vi "BuildThermomechanicalStave-Old.vi"() -> ()   [LabVIEW 2016]
doc: "This VI is the overarching framework for the ITk Stave Assembly at Brookhaven National Lab. This VI coordinates all SubVIs so that the user can execute all phases of construction: Calibration, Module Placement, and Final Survey. Learn more at https://github.com/sciollalab/BNL_ThermomechanicalStave/wiki"
uses:
  <vilib>/userdefined/High Color/IMAQdx.ctl
  Utils/Controls/All_Enums/Enum_TypeDef_CameraCalibrationResults.ctl
  Utils/Controls/0_XYZstage/DoHomeControl.ctl
  <vilib>/vision/Image Controls.llb/IMAQ Image.ctl
  C:/Users/Aerotech/Documents/BNLStaveAssembly-blueprint/Bin/Aerotech.A3200.dll
  BNLStaveAssembly-blueprint/Bin/Aerotech.A3200.dll
  Utils/Controls/0_XYZstage/BOOL_Moving.ctl
  Utils/Controls/0_XYZstage/CurrentMonitoring.ctl
  Utils/Controls/0_XYZstage/CurrentPositionReader.ctl
  Utils/Controls/0_XYZstage/SpeedReader.ctl
  Utils/Controls/0_XYZstage/BOOLs_AxesEnabled.ctl
  Utils/Controls/0_XYZstage/JogControlPanel.ctl
  Utils/Controls/All_Enums/Enum_TypeDef_JogStepSize.ctl
  Utils/Controls/BuildConfig.ctl
  Utils/Controls/All_Enums/Enum_TypeDef_TapeType.ctl
  Utils/Controls/All_Enums/Enum_TypeDef_StaveCalibMethod.ctl
  Utils/Controls/All_Enums/Enum_TypeDef_FidMarkers.ctl
  Utils/Controls/All_Enums/Enum_TypeDef_Sensors.ctl
  Utils/Controls/All_Enums/Enum_TypeDef_ImageSharpnessAnalysisMethod.ctl
  Utils/Controls/All_Enums/Ring_TypeDef_PixUmConversionMethod.ctl
  <vilib>/Analysis/coordinate.llb/2D Cartesian Coordinate Shift (Scalar).vi
  <vilib>/Utility/file.llb/Write Delimited Spreadsheet (DBL).vi
  <vilib>/vision/driver/NI_Vision_Acquisition_Software.lvlib
  <vilib>/Analysis/NI_AALPro.lvlib
  <vilib>/LabVIEW Interface for Arduino/LabVIEW Interface for Arduino.lvlib
panel:
  in  "OK Button":bool
  out "Thermometer [C]":dbl(slide)=23.623287584180844 scale=0.0..50.0
  in  "Spotlights":bool
  in  "Coaxial light":bool=TRUE
  out "Bus tape circle":cluster{"X":dbl, "Y":dbl, "Z":dbl}={"X"=-450.31300021754697, "Y"=123.45400422644629, "Z"=16.499993498862505}
  out "Calibration Type":u16(ring) items=["Bus Tape", "Tooling Pin", "Quick Calib"]
  in  "Quick Calib?":bool
  out "Camera Gain Autofocus":dbl
  out "Stave ID":string="NewDayHopePrevails"
  out "double( Time, Temp )":dbl[](array[numeric])=[12.0, 37.0, 35.0, 0.391695499420166, 23.623287584180844]
  out "VISA error out":errorcluster
  out "Camera error out":errorcluster={"status"=FALSE, "code"=1073676294, "source"="VISA Read in LabVIEW Interface for Arduino.lvlib:Send Receive.vi->LabVIEW Interface for Arduino.lvlib:Analog Read Pin.vi->LabVIEW Interface for Arduino.lvlib:Thermistor Read.vi->ArduinoLT_Config.vi->BuildThermomechanicalStave.vi"}
  in  "Abort stage":bool
  in  "Tab Control: Stave Maps":T1(tab)
  out "Module fiducials in the XYZ stage's basis":T2(graph)=[{"Generated List of Module Coordinates"=[-645.0722656433512, 536.3626218584878], "Generated List of Module Coordinates"=[124.24939561143826, 124.02687149848252]}, {"Generated List of Module Coordinates"=[-641.8178604002132, -546.3378692422014, -546.2960561473427, -641.7760473053545, -543.8178694755677, -448.3378783175558, -448.29606522269717, -543.776056380709, -445.81787855092205, -350.33788739291026, -350.2960742980516, -445.7760654560634, -347.8178876262765, -252.33789646826466, -252.29608337340602, -347.77607453141786, -249.81789670163096, -154.33790554361912, -154.29609244876048, -249.77608360677232, -151.8179057769854, -56.33791461897363, -56.29610152411499, -151.77609268212677, -53.81791485233987, 41.66207630567192, 41.70388940053056, -53.77610175748123, 44.18207607230568, 139.66206723031758, 139.70388032517621, 44.223889167164316, 142.18206699695122, 237.66205815496312, 237.70387124982176, 142.22388009180986, 240.18205792159688, 335.66204907960866, 335.7038621744673, 240.22387101645552, 338.1820488462424, 433.6620400042543, 433.7038530991131, 338.22386194110106, 436.18203977088797, 531.6620309288999, 531.7038440237586, 436.2238528657467, 534.1820306955335, 629.6620218535454, 629.7038349484042, 534.2238437903923], "Generated List of Module Coordinates"=[149.567836243492, 149.52674529578715, 246.6847362984067, 246.72582724611155, 149.52566078397092, 149.48456983626608, 246.64256083888563, 246.68365178659045, 149.48348532444982, 149.442394376745, 246.60038537936455, 246.64147632706937, 149.44130986492874, 149.4002189172239, 246.55820991984345, 246.5993008675483, 149.39913440540764, 149.35804345770282, 246.51603446032235, 246.5571254080272, 149.35695894588656, 149.31586799818172, 246.47385900080127, 246.51494994850609, 149.31478348636546, 149.27369253866064, 246.4316835412802, 246.472774488985, 149.27260802684438, 149.23151707913954, 246.3895080817591, 246.43059902946393, 149.23043256732328, 149.18934161961846, 246.347332622238, 246.38842356994283, 149.1882571078022, 149.14716616009736, 246.30515716271694, 246.34624811042175, 149.14608164828113, 149.10499070057628, 246.26298170319583, 246.30407265090068, 149.10390618876002, 149.0628152410552, 246.22080624367473, 246.26189719137957, 149.06173072923895, 149.0206397815341, 246.17863078415365, 246.21972173185847]}, {"Generated List of Module Coordinates"=[-594.056958273778, -496.05696734913244, -398.05697642448683, -300.0569854998413, -202.05699457519572, -104.0570036505502, -6.057012725904656, 91.94297819874095, 189.9429691233865, 287.9429600480321, 385.94295097267775, 483.9429418973233, 581.9429328219688], "Generated List of Module Coordinates"=[198.12628627094935, 198.08411081142827, 198.04193535190717, 197.9997598923861, 197.957584432865, 197.91540897334392, 197.8732335138228, 197.83105805430174, 197.78888259478066, 197.74670713525956, 197.70453167573848, 197.66235621621738, 197.6201807566963]}]
  out "Module Progress Report":T3(array[cluster])=[{"B"=FALSE, "A"=FALSE, "D"=FALSE, "C"=FALSE, "ID"="", "Module #"=1, "x, centre"=-594.056958273778, "y, centre"=198.12628627094935, "Aligned"=FALSE, "Glue applied"=FALSE, "Placed"=FALSE}, {"B"=FALSE, "A"=FALSE, "D"=FALSE, "C"=FALSE, "ID"="", "Module #"=2, "x, centre"=-496.05696734913244, "y, centre"=198.08411081142827, "Aligned"=FALSE, "Glue applied"=FALSE, "Placed"=FALSE}, {"B"=FALSE, "A"=FALSE, "D"=FALSE, "C"=FALSE, "ID"="", "Module #"=3, "x, centre"=-398.05697642448683, "y, centre"=198.04193535190717, "Aligned"=FALSE, "Glue applied"=FALSE, "Placed"=FALSE}, {"B"=FALSE, "A"=FALSE, "D"=FALSE, "C"=FALSE, "ID"="", "Module #"=4, "x, centre"=-300.0569854998413, "y, centre"=197.9997598923861, "Aligned"=FALSE, "Glue applied"=FALSE, "Placed"=FALSE}, {"B"=FALSE, "A"=FALSE, "D"=FALSE, "C"=FALSE, "ID"="", "Module #"=5, "x, centre"=-202.05699457519572, "y, centre"=197.957584432865, "Aligned"=FALSE, "Glue applied"=FALSE, "Placed"=FALSE}, {"B"=FALSE, "A"=FALSE, "D"=FALSE, "C"=FALSE, "ID"="", "Module #"=6, "x, centre"=-104.0570036505502, "y, centre"=197.91540897334392, "Aligned"=FALSE, "Glue applied"=FALSE, "Placed"=FALSE}, {"B"=FALSE, "A"=FALSE, "D"=FALSE, "C"=FALSE, "ID"="", "Module #"=7, "x, centre"=-6.057012725904656, "y, centre"=197.8732335138228, "Aligned"=FALSE, "Glue applied"=FALSE, "Placed"=FALSE}, {"B"=FALSE, "A"=FALSE, "D"=FALSE, "C"=FALSE, "ID"="", "Module #"=8, "x, centre"=91.94297819874095, "y, centre"=197.83105805430174, "Aligned"=FALSE, "Glue applied"=FALSE, "Placed"=FALSE}, {"B"=FALSE, "A"=FALSE, "D"=FALSE, "C"=FALSE, "ID"="", "Module #"=9, "x, centre"=189.9429691233865, "y, centre"=197.78888259478066, "Aligned"=FALSE, "Glue applied"=FALSE, "Placed"=FALSE}, {"B"=FALSE, "A"=FALSE, "D"=FALSE, "C"=FALSE, "ID"="", "Module #"=10, "x, centre"=287.9429600480321, "y, centre"=197.74670713525956, "Aligned"=FALSE, "Glue applied"=FALSE, "Placed"=FALSE}, {"B"=FALSE, "A"=FALSE, "D"=FALSE, "C"=FALSE, "ID"="", "Module #"=11, "x, centre"=385.94295097267775, "y, centre"=197.70453167573848, "Aligned"=FALSE, "Glue applied"=FALSE, "Placed"=FALSE}, {"B"=FALSE, "A"=FALSE, "D"=FALSE, "C"=FALSE, "ID"="", "Module #"=12, "x, centre"=483.9429418973233, "y, centre"=197.66235621621738, "Aligned"=FALSE, "Glue applied"=FALSE, "Placed"=FALSE}, {"B"=FALSE, "A"=FALSE, "D"=FALSE, "C"=FALSE, "ID"="", "Module #"=13, "x, centre"=581.9429328219688, "y, centre"=197.6201807566963, "Aligned"=FALSE, "Glue applied"=FALSE, "Placed"=FALSE}]
  in  "Tab Control: Config and Calib":enum32{"Configuration", "Calibration"}(tab)=enum."Calibration"
  out "Stave Orientation":bool
  in  "Code path":path=path "C:/Users/Aerotech/Documents/BNL_ThermomechanicalStave"
  in  "Reports path":path
  in  "Build Config":T4={"Tape Type"=enum."Stereo (Sutcliffe 21-Jun-18- Electrical)", "Stave Coordinate System"=enum."Bus Tape", "Module fiducial marker"=enum."Mark E (Slim/17)", "N Modules"=13}
  in  "Camera Name":T8="cam1" caption="IMAQdx Session"
  in  "Wait time before \nimage capture [s]":dbl=3.5
  in  "Placement tolerance [um]":dbl=25.0
  in  "Home stage?":T9
  in  "Sensor Pattern":T10=enum."ATLAS12Slim"
  out "Strip pitch [um]":dbl=74.5
  out "Image Collection Progress":u8(slide)=2 scale=0.0..2.0
  in  "Camera working distance scan":T11={"Stepsize [mm]"=0.2, "Focusing test interval [mm]"=2.0} {"Focusing test interval [mm]" format="%#_13g"}
  in  "XYZ Stage Frame: Coordinates for calibration":T12={"Stave Origin"={"X [mm]"=-644.095, "Y [mm]"=133.592, "Z [mm]"=14.999958}, "Cam calib"={"X [mm]"=-554.0949106430569, "Y [mm]"=73.59263357310083, "Z [mm]"=16.5}, "Bus Tape Circle"={"X [mm]"=-479.095, "Y [mm]"=123.592, "Z [mm]"=16.499993500000002}}
  out "Calibration Results":T14={"Camera calibration results"={"Working distance to stave [mm]"=0.0, "WD Uncertainty [mm]"=0.0, "Calibration [um/pix]"=0.0, "Calib uncertainty [um/pix]"=0.0}, "Stave basis calibration results"={"Angle, stave & xyz stage [rad]"=0.0, "Calibrated stave origin (X,Y) [mm]"=[-450.33678692531066, 123.45352825130794]}} {"Camera calibration results"."Working distance to stave [mm]" format="%#_13g"}
  in  "Jogging Controls":T15={"Jog step size"={"X [mm]"=enum."1 mm", "Y [mm]"=enum."1 mm", "Z [mm]"=enum."[None]"}, "Left"=FALSE, "Right"=FALSE, "Forward"=FALSE, "Backward"=FALSE, "Up"=FALSE, "Down"=FALSE, "Reset position"=FALSE, "Confirm position"=FALSE}
  out "BUILD STAVE: STATUS REPORT":T22={"Current Build Phase"="Positioning modules on the Axial (Sutcliffe NP49-01-100 01-Mar-16) side: Consult VisualizingModulePositions front panel... ", "Completion Status"={"Calibrated? "={"Stage homed"=TRUE, "Camera height"=TRUE, "Pix/um"=TRUE, "Stave basis"=TRUE}, "Mounted?"={"Virtual stave"=TRUE, "Processing module #"=""}, "Surveyed?"={"Before curing"=FALSE, "After curing"=FALSE}}, "Current time and temperature"=["6/22/2018 12:37:35 PM", "23.623288"], "Moving"=FALSE, "Current monitoring"={{"X Current Cmd [A]"=0.06695456, "Y Current Cmd [A]"=0.4440778, "Z Current Cmd [A]"=-0.28503352}, {"X Current Feedback [A]"=0.0660152, "Y Current Feedback [A]"=0.44387716, "Z Current Feedback [A]"=-0.28616208}}, "Current stage position [mm]"={"X"=529.9771835386682, "Y"=123.87540176748969, "Z"=18.805003718415485}, "Axis Speeds [mm/s]"={"X"=45.0, "Y"=25.0, "Z"=25.0}, "Axes enabled?"={"X"=TRUE, "Y "=TRUE, "Z"=TRUE}}
  out "Reset coordinates":cluster{"X":dbl, "Y":dbl, "Z":dbl}={"X"=-450.3131879006525, "Y"=123.45397637915625, "Z"=16.499993498862505}
  out "Image collection inputs":T24={"Current field of view"="remote image 000000000F72BDBC", "Axis Speeds"={"X [mm/s]"=45.0, "Y [mm/s]"=25.0, "Z [mm/s]"=25.0}, "XYZ Stage Control"=refnum}
  in  "Camera gain":dbl
  out "Wait to capture [ms]":u32=3500
  out "Baseline Z [mm]":dbl=16.499993498862505
  out "Calibrated module height":dbl=16.701535010654045
  out "Calibrated stave basis [mm]":dbl[][](array[numeric])=[[-450.33678692531066, 123.45352825130794, 18.80496998830317], [529.977188416502, 123.87541800859147, 18.80496998830317]]
  out "Camera calibration pattern":T25={"X [mm]"=580.0001203076404, "Y [mm]"=68.99983358489945, "Z [mm]"=16.499993498862505}
  out "Stave origin":T25={"X [mm]"=-630.6520112612299, "Y [mm]"=126.45397794714735, "Z [mm]"=14.999958002771999}
  out "Focusing test interval [mm]":dbl=3.0
  out "Stepsize [mm]":dbl=0.2
  out "delta Z":dbl=-0.20154151179153956
  out "Calibrated stave origin (X,Y) [mm]":dbl[](array[numeric])=[-450.33678692531066, 123.45352825130794]
  out "Angle between stave and xyz stage":dbl=0.00043036184513248925
  out "Average microns/pixel":ext
  out "Optimized Z [mm]":dbl=16.701535010654045 format="%#_13g"
  out "Current field of view":T23(plugin-control)
  in  "Program Errors":errorcluster={"status"=FALSE, "code"=1073676294, "source"="VISA Read in LabVIEW Interface for Arduino.lvlib:Send Receive.vi->LabVIEW Interface for Arduino.lvlib:Analog Read Pin.vi->LabVIEW Interface for Arduino.lvlib:Thermistor Read.vi->ArduinoLT_Config.vi->BuildThermomechanicalStave.vi"}
  # "BUILD THERMOMECHANICAL STAVE Brandeis University - Brookhaven National Laboratory * ATLAS Phase II Inner Tracker Upgrade\nAuthors: L. Bergsten, P. Bhattarai, A. Garcia, H. Herde, C. Nicoloff, G. Sciolla"
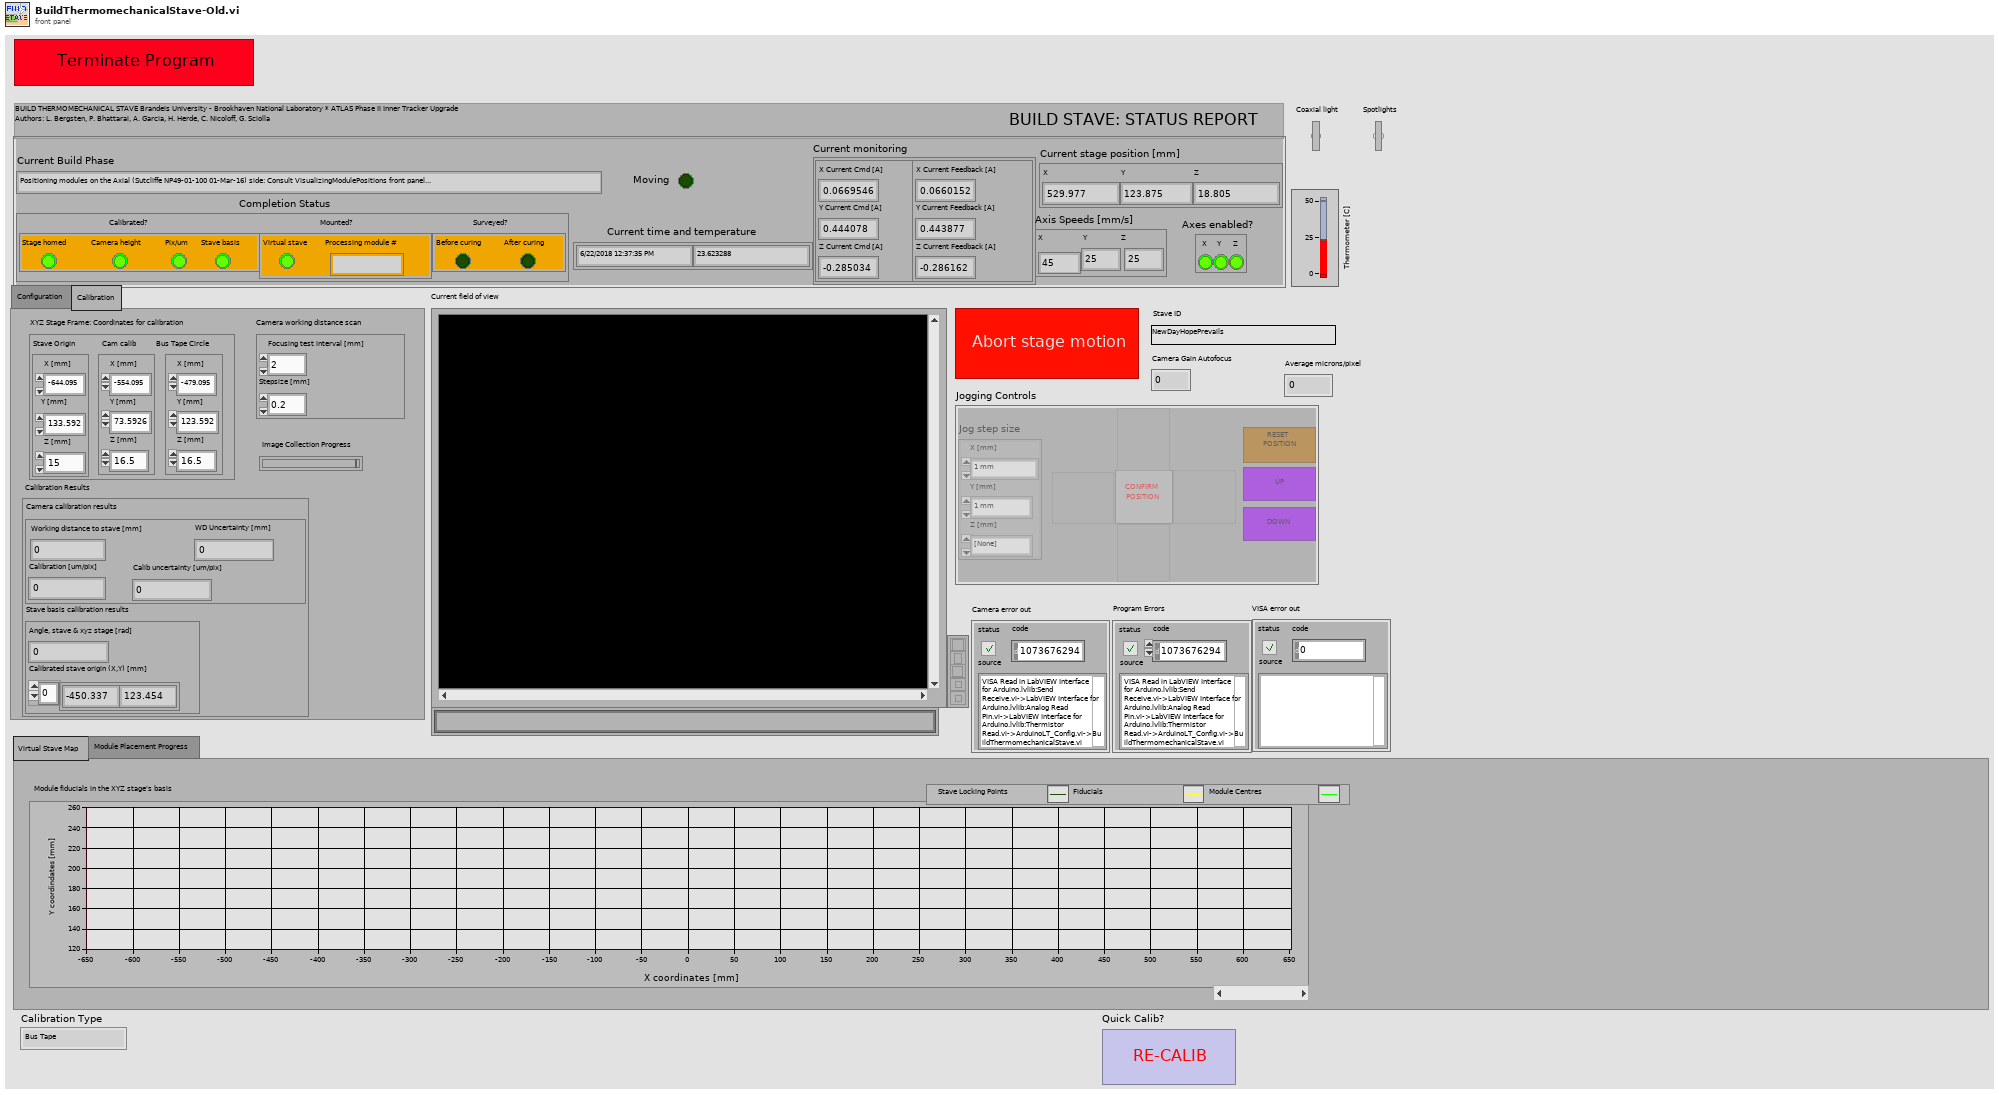
[diagram p1: front panel]
types:
  T1 = enum32{"Virtual Stave Map", "Module Placement Progress"}
  T2 = cluster{"Generated List of Module Coordinates":dbl[], "Generated List of Module Coordinates":dbl[]}[]
  T3 = cluster{"B":bool, "A":bool, "D":bool, "C":bool, "ID":string, "Module #":i32, "x, centre":dbl, "y, centre":dbl, "Aligned":bool, "Glue applied":bool, "Placed":bool}[]
  T4 = typedef "BuildConfig.ctl" = cluster{"Tape Type":T5, "Stave Coordinate System":T6, "Module fiducial marker":T7, "N Modules":i32}
  T5 = typedef "Enum_TypeDef_TapeType.ctl" = enum16{"Right stereo", "Left stereo", "Stereo (Sutcliffe NP49-01-100 01-Mar-16)", "Stereo (Sutcliffe 21-Jun-18- Electrical)", "Axial (Sutcliffe NP49-01-100 01-Mar-16)"}
  T6 = typedef "Enum_TypeDef_StaveCalibMethod.ctl" = enum16{"Tooling Pins", "Bus Tape"}
  T7 = typedef "Enum_TypeDef_FidMarkers.ctl" = enum16{"Mark B", "Mark C", "Bias Ring Corner", "Mark I (Slim/17)", "Mark E (Slim/17)", "Mark F (Slim/17)", "Mark G (Slim/17)", "Mark A (12)", "Kapton Spacers"}
  T8 = typedef "IMAQdx.ctl" = refnum<k21>
  T9 = typedef "DoHomeControl.ctl" = bool
  T10 = typedef "Enum_TypeDef_Sensors.ctl" = enum16{"ATLAS07", "ATLAS12", "ATLAS12Slim", "ATLAS17LS"}
  T11 = cluster{"Stepsize [mm]":dbl, "Focusing test interval [mm]":dbl}
  T12 = cluster{"Stave Origin":cluster{"X [mm]":dbl, "Y [mm]":dbl, "Z [mm]":dbl}, "Cam calib":cluster{"X [mm]":dbl, "Y [mm]":dbl, "Z [mm]":dbl}, "Bus Tape Circle":cluster{"X [mm]":dbl, "Y [mm]":dbl, "Z [mm]":dbl}}
  T13 = typedef "Enum_TypeDef_CameraCalibrationResults.ctl" = cluster{"Working distance to stave [mm]":dbl, "WD Uncertainty [mm]":dbl, "Calibration [um/pix]":dbl, "Calib uncertainty [um/pix]":dbl}
  T14 = cluster{"Camera calibration results":T13, "Stave basis calibration results":cluster{"Angle, stave & xyz stage [rad]":dbl, "Calibrated stave origin (X,Y) [mm]":dbl[]}}
  T15 = typedef "JogControlPanel.ctl" = cluster{"Jog step size":T16, "Left":bool, "Right":bool, "Forward":bool, "Backward":bool, "Up":bool, "Down":bool, "Reset position":bool, "Confirm position":bool}
  T16 = typedef "Enum_TypeDef_JogStepSize.ctl" = cluster{"X [mm]":enum16{"1 um", "5 um", "10 um", "0.1 mm", "0.25 mm", "0.5 mm", "1 mm", "5 mm", "10 mm", "20 mm", "50 mm"}, "Y [mm]":enum16{"1 um", "5 um", "10 um", "0.1 mm", "0.25 mm", "0.5 mm", "1 mm", "5 mm", "10 mm", "20 mm", "50 mm"}, "Z [mm]":enum16{"1 um", "5 um", "10 um", "0.1 mm", "0.25 mm", "0.5 mm", "1 mm", "5 mm", "10 mm", "20 mm", "[None]"}}
  T17 = typedef "BOOL_Moving.ctl" = bool
  T18 = typedef "CurrentMonitoring.ctl" = cluster{cluster{"X Current Cmd [A]":sgl, "Y Current Cmd [A]":sgl, "Z Current Cmd [A]":sgl}, cluster{"X Current Feedback [A]":sgl, "Y Current Feedback [A]":sgl, "Z Current Feedback [A]":sgl}}
  T19 = typedef "CurrentPositionReader.ctl" = cluster{"X":dbl, "Y":dbl, "Z":dbl}
  T20 = typedef "SpeedReader.ctl" = cluster{"X":dbl, "Y":dbl, "Z":dbl}
  T21 = typedef "BOOLs_AxesEnabled.ctl" = cluster{"X":bool, "Y ":bool, "Z":bool}
  T22 = cluster{"Current Build Phase":string, "Completion Status":cluster{"Calibrated? ":cluster{"Stage homed":bool, "Camera height":bool, "Pix/um":bool, "Stave basis":bool}, "Mounted?":cluster{"Virtual stave":bool, "Processing module #":string}, "Surveyed?":cluster{"Before curing":bool, "After curing":bool}}, "Current time and temperature":string[], "Moving":T17, "Current monitoring":T18, "Current stage position [mm]":T19, "Axis Speeds [mm/s]":T20, "Axes enabled?":T21}
  T23 = typedef "IMAQ Image.ctl" = refnum<image>
  T24 = cluster{"Current field of view":T23, "Axis Speeds":cluster{"X [mm/s]":dbl, "Y [mm/s]":dbl, "Z [mm/s]":dbl}, "XYZ Stage Control":refnum<k24>}
  T25 = cluster{"X [mm]":dbl, "Y [mm]":dbl, "Z [mm]":dbl}
  T26 = cluster{"Current Build Phase":string, "Completion Status":cluster{"Calibrated? ":cluster{"Stage homed":bool, "Camera height":bool, "pix/um":bool, "Stave basis":bool}, "Mounted?":cluster{"Virtual stave":bool, "Current module #":string}, "Surveyed?":cluster{"Before curing":bool, "After curing":bool}}, "Current time and temperature":string[], "Moving":bool, "Current monitoring":cluster{cluster{"X Current Cmd [A]":sgl, "Y Current Cmd [A]":sgl, "Z Current Cmd [A]":sgl}, cluster{"X Current Feedback [A]":sgl, "Y Current Feedback [A]":sgl, "Z Current Feedback [A]":sgl}}, "Current stage position [mm]":cluster{"X":dbl, "Y":dbl, "Z":dbl}, "Axis Speeds [mm/s]":cluster{"X":dbl, "Y":dbl, "Z":dbl}, "Axes enabled?":cluster{"X":bool, "Y ":bool, "Z":bool}}
  T27 = enum8{"Enabled", "Disabled", "Disabled and Grayed Out"}
  T28 = cluster{"Camera calibration results":cluster{"Calibration [um/pix]":dbl, "Working distance to stave [mm]":dbl, "Calib uncertainty [um/pix]":dbl, "WD Uncertainty [mm]":dbl}, "Stave basis calibration results":cluster{"Angle, stave & xyz stage [rad]":dbl, "Calibrated stave origin (X,Y) [mm]":dbl[]}}
  T29 = typedef "Image Type" = u32
  T30 = typedef "LabVIEW Interface for Arduino.lvlib/Arduino Resource.ctl" = cluster{"VISA resource":refnum<visa-resource-name>, "Board Type":T31, "Connection Type":enum8{"USB / Serial"}, "Bytes Per Packet (15)":u8}
  T31 = typedef "LabVIEW Interface for Arduino.lvlib/Board Type.ctl" = enum16{"Uno", "Dimuelanove w/Atmega 328", "Mega 2560"}
  T32 = typedef "ArduinoLT-ConfigurationControl.ctl" = cluster{"Lights: Digital I/O Pins":cluster{"Coaxial":u8, "Spotlights":u8}, "Thermistor Settings":cluster{"Analogue Readout Pin":u8, "Vcc Reference Pin":u8, "Paired Resistance (10K Ohms)":dbl, "Units (C)":enum16{"Celsius", "Fahrenheit", "Kelvin"}}}
  T33 = cluster{"Camera session out":T8, "New Image":T23}
  T34 = cluster{cluster{"X Current Cmd [A]":sgl, "Y Current Cmd [A]":sgl, "Z Current Cmd [A]":sgl}, cluster{"X Current Feedback [A]":sgl, "Y Current Feedback [A]":sgl, "Z Current Feedback [A]":sgl}}
  T35 = cluster{"X [mm]":dbl, "Y [mm]":dbl, "Z [mm]":dbl}[]
  T36 = cluster{"Final X":dbl, "Final Y":dbl, "Final Z":dbl}
  T37 = cluster{"Step size [mm]":dbl, "Step size [mm]":dbl, "Step size [mm]":dbl}
  T38 = cluster{"[0]":cluster{"X":dbl, "Y":dbl, "Z":dbl}, "[1]":cluster{"X":dbl, "Y":dbl, "Z":dbl}, "[2]":cluster{"X":dbl, "Y":dbl, "Z":dbl}}
  T39 = typedef "Enum_TypeDef_ImageSharpnessAnalysisMethod.ctl" = enum16{"sigma( Intensity )", "Mean( Laplacian Convolution )"}
  T40 = typedef "Ring_TypeDef_PixUmConversionMethod.ctl" = u16
  T41 = cluster{"Current field of view":T23, "Value":cluster{"X":dbl, "Y":dbl, "Z":dbl}, "Aerotech out":refnum<k24>}
  T42 = cluster{"Captured positions":dbl[][], "XYZ .NET Refnum out":refnum<k24>}
  T43 = cluster{"Calibrated stave basis [mm]":dbl[], "Calibrated stave basis [mm]":dbl[]}
  T44 = cluster{"Calibrated stave basis [mm]":dbl[], "Calibrated stave basis [mm]":dbl[]}[]
diagram:
  w51 = u32 15705600 ("Color")
  w95 = errorcluster {"status"=FALSE, "code"=0, "source"=""}  # VISA Errors
  w78 = errorcluster {"status"=FALSE, "code"=0, "source"=""}  # Camera Errors
  w52 = T26 {"Current Build Phase"="Welcome, Stave Builder!", "Completion Status"={"Calibrated? "={"Stage homed"=FALSE, "Camera height"=FALSE, "pix/um"=FALSE, "Stave basis"=FALSE}, "Mounted?"={"Virtual stave"=FALSE, "Current module #"=""}, "Surveyed?"={"Before curing"=FALSE, "After curing"=FALSE}}, "Current time and temperature"=[], "Moving"=FALSE, "Current monitoring"={{"X Current Cmd [A]"=0.0, "Y Current Cmd [A]"=0.0, "Z Current Cmd [A]"=0.0}, {"X Current Feedback [A]"=0.0, "Y Current Feedback [A]"=0.0, "Z Current Feedback [A]"=0.0}}, "Current stage position [mm]"={"X"=0.0, "Y"=0.0, "Z"=0.0}, "Axis Speeds [mm/s]"={"X"=45.0, "Y"=25.0, "Z"=25.0}, "Axes enabled?"={"X"=FALSE, "Y "=FALSE, "Z"=FALSE}}  # BUILD STAVE: STATUS REPORT
  w50 = FALSE ("Left")
  w49 = T27."Disabled and Grayed Out" ("Disabled")
  w187 = TRUE ("Calibrated?")
  w194 = u32 16761088 ("Color")
  w203 = T29 0 items=["Grayscale (U8)", "Grayscale (I16)", "Grayscale (SGL)", "Complex (CSG)", "RGB (U32)", "HSL (U32)", "RGB (U64)", "Grayscale (U16)"] ("Image Type")
  n1 = property on="Sensor Pattern" class="Enum (strict)"() -> ("Strings []"=w8:string[])  [unwired: 2 in, 2 out]
  n2 = Index Array(array=w8, index="Sensor Pattern") -> (element=w7:string)
  n3 = Concatenate Strings(w7, ".ini" ("string")) -> (w11:string)
  n4 = Build Path(base path="Code path", name or relative path="Utils\\ConfigurationFiles_and_Templates\\1_ModulePlacement\\0_ModuleLayouts") -> (appended path=w10:path)
  n5 = Build Path "Select configuration file"(base path=w10, name or relative path=w11) -> (appended path=w5:path)
  n6 = call "ReadModuleConfiguration (SubVI).vi"("Module configuration file path"=w5) -> ("Strip pitch [um]"=→"Strip pitch [um]":dbl)  [unwired: 8 in, 6 out]
  n7 = disable-structure shown="Disabled" {
    frame Disabled {
      n8 = local read "Calibrated stave origin (X,Y) [mm]"() -> ()  [unwired: 1 out]
    }
    frame Enabled {
    }
  }
  n9 = local write "Module fiducials in the XYZ stage's basis"(T2 [{"Generated List of Module Coordinates"=[], "Generated List of Module Coordinates"=[]}, {"Generated List of Module Coordinates"=[-299.2110287057527, -202.7315011933668, -202.42767808647434, -298.9072055988603, -201.21150863720152, -104.73198112481558, -104.42815801792312, -200.90768553030907, -103.2119885686503, -6.732461056264299, -6.4286379493718755, -102.90816546175785, -5.212468500099078, 91.2670590122869, 91.57088211917932, -4.908645393206655, 92.78705156845217, 189.26657908083814, 189.57040218773056, 93.0908746753446, 190.7865716370033, 287.2660991493893, 287.5699222562817, 191.09039474389573, 288.7860917055545, 385.26561921794047, 385.5694423248329, 289.0899148124469, 386.7856117741057, 483.26513928649166, 483.5689623933841, 387.0894348809981, 484.7851318426569, 581.2646593550428, 581.5684824619352, 485.0889549495493, 582.7846519112081, 679.264179423594, 679.5680025304864, 583.0884750181006, 680.7841719797593, 777.2636994921454, 777.5675225990378, 681.0879950866517, 778.7836920483107, 875.2632195606966, 875.567042667589, 779.0875151552032, 876.7832121168619, 973.2627396292478, 973.5665627361402, 877.0870352237544], "Generated List of Module Coordinates"=[18.614201133837582, 18.312255796456228, 115.39178037048637, 115.69372570786773, 18.307498780361485, 18.00555344298013, 115.08507801701028, 115.38702335439163, 18.0007964268854, 17.698851089504046, 114.77837566353418, 115.08032100091555, 17.694094073409303, 17.39214873602795, 114.4716733100581, 114.77361864743946, 17.38739171993322, 17.08544638255185, 114.16497095658201, 114.46691629396337, 17.080689366457122, 16.778744029075767, 113.85826860310591, 114.16021394048727, 16.77398701298104, 16.47204167559967, 113.55156624962981, 113.85351158701118, 16.46728465950494, 16.165339322123586, 113.24486389615373, 113.54680923353509, 16.160582306028857, 15.858636968647488, 112.93816154267763, 113.240106880059, 15.85387995255276, 15.551934615171405, 112.63145918920155, 112.9334045265829, 15.547177599076676, 15.245232261695307, 112.32475683572545, 112.62670217310682, 15.240475245600578, 14.938529908219223, 112.01805448224937, 112.31999981963072, 14.933772892124495, 14.631827554743126, 111.71135212877327, 112.01329746615463]}, {"Generated List of Module Coordinates"=[-250.8193533961135, -152.81983332756232, -54.82031325901109, 43.17920680954012, 141.17872687809137, 239.1782469466425, 337.1777670151937, 435.1772870837449, 533.1768071522961, 631.1763272208473, 729.1758472893986, 827.1753673579499, 925.1748874265011], "Generated List of Module Coordinates"=[67.00299075216198, 66.69628839868588, 66.3895860452098, 66.0828836917337, 65.77618133825762, 65.46947898478152, 65.16277663130543, 64.85607427782934, 64.54937192435324, 64.24266957087715, 63.935967217401064, 63.62926486392497, 63.32256251044888]}] ("Module fiducials in the XYZ stage's basis")) -> ()
  n10 = property on="Calibrated?" class="Clust (strict)"(error in=w78, "Color"=w194) -> (error out=w130:errorcluster)  [unwired: 1 in, 1 out]
  n11 = property on="Mounted?" class="Clust (strict)"(error in=w78, "Color"=w194) -> (error out=w129:errorcluster)  [unwired: 1 in, 1 out]
  n12 = property on="Surveyed?" class="Clust (strict)"(error in=w78, "Color"=w194) -> (error out=w128:errorcluster)  [unwired: 1 in, 1 out]
  n13 = property on="Calibrated?" class="Clust (strict)"("Color"=w51) -> ()  [unwired: 2 in, 2 out]
  n14 = property on="Surveyed?" class="Clust (strict)"("Color"=w51) -> ()  [unwired: 2 in, 2 out]
  n15 = property on="Mounted?" class="Clust (strict)"("Color"=w51) -> ()  [unwired: 2 in, 2 out]
  n16 = Merge Errors(w130, w129, w128) -> (w45:errorcluster)
  n17 = call "ArduinoLT_Config.vi"("error in"=w45, "VISA resource"=refnum<visa-resource-name> "LightsCTRL") -> ("error out"=w40:errorcluster, "Arduino Resource"=w14:T30, "Arduino Configuration OUT"=w19:T32)  [unwired: 3 in, 1 out]
  n18 = control-ref of="Spotlights"() -> (w42:refnum<vi>)
  n19 = control-ref of="Coaxial light"() -> (w43:refnum<vi>)
  n20 = call "CheckLightingConditions.vi"("Bus Tape Gain"=16.0, "Change Lights? (Change; Coax; Spotlight)"=bool[] [TRUE, TRUE, TRUE], "Si Gain"=2.0, "error in (no error)"=w40, "Spotlights Refnum"=w42, "Coaxial Lights Refnum"=w43) -> ("error out"=w41:errorcluster, "Assigned Camera Gain"=w36:dbl)  [unwired: 2 in, 2 out]
  n21 = while "Monitor time and temperature/ Stops the VI if button pressed" {
    tunnel: w95 -> [w211]
    tunnel: w19 -> [w209]
    tunnel: [w210] -> w18
    tunnel: [w208] -> w17
    tunnel: [w208] -> w15
    tunnel: w14 -> [w207]
    stop <- w212 stop-if-true
    n22 = case shown="True" "OK Button" {
      tunnel: [w230 w235] -> w212
      tunnel: w211 -> [w220 w237]
      tunnel: [w219 w236] -> w210
      tunnel: w209 -> [w218 _]
      tunnel: [w214 w234] -> w208
      tunnel: w207 -> [w213 w236]
      frame False {
        n23 = call "ArduinoLT_Collect_Control.vi"("Arduino Configuration"=w218, "error in"=w220, "Arduino Resource IN"=w213, "Spotlights"="Spotlights", "Coaxial light"="Coaxial light") -> ("error out"=w222:errorcluster, "Arduino Resource OUT"=w219:T30, "Thermometer [C]"=w221:dbl)  [unwired: 4 in]
        "Thermometer [C]" <- w221
        n24 = Wait (ms)(milliseconds to wait=u32 500) -> ()  [unwired: 1 out]
        n25 = call "ArduinoLT-TimeAndTempature.vi"("error in (no error)"=w222, "Temperature"=w221) -> ("error out"=w224:errorcluster, "double( Time, Temp )"=→"double( Time, Temp )":dbl[], "str( Time, Temp )"=w215:string[])  [unwired: 7 in]
        n26 = property on="Current time and temperature" class="Arr (strict)"(error in=w224, "Value"=w215) -> (error out=w229:errorcluster)  [unwired: 1 in, 1 out]
        n27 = Multiply(x="Wait time before \nimage capture [s]", y=u32 1000) -> (x*y=→"Wait to capture [ms]":dbl)
        n28 = call <vilib>:"Simple Error Handler.vi"("error in (no error)"=w229) -> ("error out"=w228:errorcluster)  [unwired: 4 in, 4 out]
        n29 = property on="After curing" class="Bool (strict)"(error in=w228) -> (error out=w214:errorcluster, "Value"=w230:bool)  [unwired: 1 in, 1 out]
      }
      frame True {
        n30 = flat-sequence {
          tunnel: w237 -> [w243]
          tunnel: w236 -> [w242]
          tunnel: [w240] -> w233
          tunnel: [w238] -> w232
          tunnel: [w245] -> w234
          tunnel: [w246] -> w235
          tunnel: w233 -> [w246]
          tunnel: w232 -> [w245]
          frame #0 {
            n31 = call <vilib>:"Close.vi"("Arduino Resource"=w242, "error in"=w243) -> ("error out"=w239:errorcluster)  [unwired: 13 in]
            n32 = call <vilib>:"Simple Error Handler.vi"("error in (no error)"=w239) -> ("error out"=w241:errorcluster)  [unwired: 4 in, 4 out]
            n33 = property on="After curing" class="Bool (strict)"(error in=w241) -> (error out=w238:errorcluster, "Value"=w240:bool)  [unwired: 1 in, 1 out]
          }
          frame #1 {
            n34 = local read "OK Button"() -> (w244:bool)
            n35 = Stop(stop? (T)=w244) -> ()
          }
        }
      }
    }
  }
  "VISA error out" <- w15
  n36 = property on="Camera gain" class="DigNum (strict)"(error in=w41, "Value"=w36) -> (error out=w20:errorcluster, "Value"=w115:dbl)  [unwired: 1 in, 1 out]
  n37 = call "IMAQ Create"("Image Name"="Grab", "Image Type"=w203, "error in (no error)"=w20) -> ("New Image"=w112:T23, "error out"=w200:errorcluster)  [unwired: 1 in, 1 out]
  n38 = call <vilib>:"IMAQdx Open Camera.vi"("error in"=w200, "Session In"="Camera Name") -> ("error out"=w201:errorcluster, "Session Out"=w204:T8)  [unwired: 1 in, 7 out]
  n39 = call <vilib>:"IMAQdx Configure Grab.vi"("error in"=w201, "Session In"=w204) -> ("error out"=w116:errorcluster, "Session Out"=w117:T8)  [unwired: 8 out]
  n40 = call "0_SetupCameraAttributes (SubVI).vi"("error in (no error)"=w116, "Gain"=w115, "Camera session in"=w117) -> ("error out"=w23:errorcluster, "Camera session out"=w113:T8)  [unwired: 7 in]
  n41 = Merge Errors("Program Errors", w23) -> (w21:errorcluster)
  n42 = case "Execute homing sequence/connect to XYZ stage and enable axes" shown="True" "Home stage?" {
    tunnel: [w250 w261] -> w127
    tunnel: [w251 w260] -> w101
    tunnel: w21 -> [w247 w255]
    frame False {
      n43 = property on="Current Build Phase" class="Str"(error in=w247, "Value"="Connecting to XYZ stage..." ("Current Build Phase")) -> (error out=w249:errorcluster)  [unwired: 1 in, 1 out]
      n44 = call "Connect.vi"("error in (no error)"=w249) -> ("error out"=w254:errorcluster, "controller"=w253:refnum<k24>)  [unwired: 9 in]
      n45 = call "EnableMultiple.vi"("error in (no error)"=w254, "axis names"=string[] ["X", "Y", "Z"] ("Axes Names"), "controller in"=w253) -> ("error out"=w250:errorcluster, "controller out"=w251:refnum<k24>)  [unwired: 7 in]
    }
    frame True {
      n46 = property on="Current Build Phase" class="Str"(error in=w255, "Value"="Homing XYZ stage..." ("Current Build Phase")) -> (error out=w258:errorcluster)  [unwired: 1 in, 1 out]
      n47 = property on="Moving" class="Bool (strict)"(error in=w258, "Value"=TRUE ("Moving")) -> (error out=w257:errorcluster)  [unwired: 1 in, 1 out]
      n48 = call "0_HomeAllAxes (SubVI).vi"("error in (no error)"=w257) -> ("error out"=w261:errorcluster, "controller out"=w260:refnum<k24>)  [unwired: 7 in, 2 out]
    }
  }
  n49 = property on="XYZ Stage Frame: Coordinates for calibration" class="Clust (strict)"(error in=w127) -> (error out=w195:errorcluster, "Controls[]"=w197:refnum<vi>[])  [unwired: 1 in, 1 out]
  n50 = Bundle("Camera session out"=w113, "New Image"=w112) -> (w111:T33)  [unwired: 1 in]
  n51 = Obtain Queue(name (unnamed)="CameraProcessing", element data type=cluster{"Session In":T8, "Image In":T23} {"Session In"="", "Image In"=refnum}, error in (no error)=w23) -> (queue out=w103:refnum<queue>, error out=w114:errorcluster)  [unwired: 2 in, 1 out]
  n52 = while "Cancel stage motion" {
    shift-right: [w262] -> _
    shift-left: w101 -> [w263]
    stop <- w264 stop-if-true
    n53 = case shown="True" "Abort stage" {
      tunnel: w263 -> [w266 w268]
      tunnel: [w266 w267] -> w262
      frame False {
      }
      frame True {
        n54 = call "AbortMultiple.vi"("axis names"=string[] ["X", "Y", "Z"], "controller in"=w268) -> ("controller out"=w267:refnum<k24>)  [unwired: 8 in, 1 out]
      }
    }
    n55 = property on="After curing" class="Bool (strict)"() -> ("Value"=w264:bool)  [unwired: 2 in, 2 out]
  }
  n56 = while "Monitor XYZ stage axes: position, motion, homing, currents" {
    tunnel: w127 -> [w273]
    shift-right: [w270] -> _
    shift-left: w101 -> [w272]
    stop <- w288 stop-if-true
    n57 = Wait (ms)(milliseconds to wait=u32 100) -> ()  [unwired: 1 out]
    n58 = call "GetStageAxesStatus (SubVI).vi"(".NET Refnum in - Device"=w272, "Axes Names"=string[] ["X", "Y", "Z"], "error in (no error)"=w273) -> ("Homed"=w287:bool, "Axis enabled"=w283:cluster{"X":bool, "Y ":bool, "Z":bool}, "Moving"=w286:bool, ".NET Refnum out  - Device"=w270:refnum<k24>, "Current stage position"=w284:T25, "Current monitoring"=w285:T34, "error out"=w275:errorcluster)  [unwired: 1 out]
    n59 = property on="Stage homed" class="Bool (strict)"(error in=w275, "Value"=w287) -> (error out=w282:errorcluster)  [unwired: 1 in, 1 out]
    n60 = property on="Moving" class="Bool (strict)"(error in=w275, "Value"=w286) -> (error out=w281:errorcluster)  [unwired: 1 in, 1 out]
    n61 = property on="Axes enabled?" class="Clust (strict)"(error in=w275, "Value"=w283) -> (error out=w280:errorcluster)  [unwired: 1 in, 1 out]
    n62 = property on="Current stage position [mm]" class="Clust (strict)"(error in=w275, "Value"=w284) -> (error out=w279:errorcluster)  [unwired: 1 in, 1 out]
    n63 = property on="Current monitoring" class="Clust (strict)"(error in=w275, "Value"=w285) -> (error out=w278:errorcluster)  [unwired: 1 in, 1 out]
    n64 = property on="After curing" class="Bool (strict)"(error in=w275) -> (error out=w276:errorcluster, "Value"=w288:bool)  [unwired: 1 in, 1 out]
    n65 = Merge Errors(w282, w281, w280, w279, w278, w276) -> (w277:errorcluster)
    n66 = call <vilib>:"Simple Error Handler.vi"("error in (no error)"=w277) -> ("error out"=w274:errorcluster)  [unwired: 4 in, 4 out]
    n67 = local write "Program Errors"(w274) -> ()
  }
  n68 = while "Consumer Loop: Constantly collect camera image" {
    shift-right: [w302] -> _
    shift-left: w103 -> [w307]
    tunnel: [w290] -> _
    stop <- w305 stop-if-true
    n69 = Dequeue Element(queue=w307) -> (queue out=w302:refnum<queue>, element=w306:cluster{"Session In":T8, "Image In":T23}, error out=w304:errorcluster)  [unwired: 2 in, 1 out]
    n70 = Unbundle By Name(w306) -> ("Session In"=w301:T8, "Image In"=w299:T23)
    n71 = call "0_SetupCameraAttributes (SubVI).vi"("error in (no error)"=w304, "Gain"="Camera gain", "Camera session in"=w301) -> ("error out"=w298:errorcluster, "Camera session out"=w300:T8)  [unwired: 7 in]
    n72 = call "AlignCameraFrame (SubVI).vi"("error in (no error)"=w298, "Image Src"=w299, "Camera session in"=w300) -> ("error out"=w292:errorcluster, "Image Dst Out"=w294:T23)  [unwired: 6 in, 1 out]
    n73 = property on="Pix/um" class="Bool (strict)"(error in=w292) -> (error out=w291:errorcluster, "Value"=w293:bool)  [unwired: 1 in, 1 out]
    n74 = case shown="True" w293 {
      tunnel: [w308 w310] -> w290
      tunnel: w294 -> [w308 w311]
      frame False {
      }
      frame True {
        n75 = local read "Average microns/pixel"() -> (w309:ext)
        n76 = call "3_DrawScale (SubVI).vi"("um/pix"=w309, "Refnum in"=w311) -> ("Refnum out"=w310:T23)  [unwired: 9 in]
      }
    }
    "Current field of view" <- w290
    n77 = call <vilib>:"Simple Error Handler.vi"("error in (no error)"=w291) -> ("error out"=w296:errorcluster)  [unwired: 4 in, 4 out]
    n78 = property on="After curing" class="Bool (strict)"(error in=w296) -> (error out=w295:errorcluster, "Value"=w303:bool)  [unwired: 1 in, 1 out]
    n79 = Compound Arithmetic op=OR(w303, w295) -> (w305:bool)
  }
  n80 = while "Producer Loop: Constantly collect camera image" {
    shift-right: [w324] -> w110
    shift-left: w103 -> [w325]
    shift-right: [w313] -> w109
    shift-left: w114 -> [w326]
    shift-right: [w315] -> w108
    shift-left: w111 -> [w318]
    stop <- w314 stop-if-true
    n81 = Unbundle By Name(w318) -> ("Camera session out"=w317:T8, "New Image"=w316:T23)
    n82 = call <vilib>:"IMAQdx Grab.vi"("error in"=w326, "Wait for Next Buffer? (Yes)"=TRUE, "Image In"=w316, "Session In"=w317) -> ("error out"=w323:errorcluster, "Image Out"=w319:T23, "Session Out"=w320:T8)  [unwired: 5 out]
    n83 = Bundle("Session Out"=w320, "Image Out"=w319) -> (w315:cluster{"Session Out":T8, "Image Out":T23})  [unwired: 1 in]
    n84 = Enqueue Element(queue=w325, element=w315, error in (no error)=w323) -> (queue out=w324:refnum<queue>, error out=w322:errorcluster)  [unwired: 1 in, 1 out]
    n85 = call <vilib>:"Simple Error Handler.vi"("error in (no error)"=w322) -> ("error?"=w328:bool, "error out"=w313:errorcluster)  [unwired: 4 in, 3 out]
    "Camera error out" <- w313
    n86 = property on="After curing" class="Bool (strict)"() -> ("Value"=w327:bool)  [unwired: 2 in, 2 out]
    n87 = Unbundle By Name(w313) -> ("status"=w321:bool)
    n88 = Compound Arithmetic op=OR(w321, w327, w328) -> (w314:bool)
  }
  n89 = Cluster To Array(cluster="XYZ Stage Frame: Coordinates for calibration") -> (array=w196:T35)
  n90 = for "Loop on calibration coordinates: jog stage to reposition camera if initial coordinate is incorrect" {
    tunnel: w196 -> [w367] mode=indexing
    tunnel: w101 -> [w368]
    tunnel: w197 -> [w363] mode=indexing
    tunnel: w195 -> [w366]
    tunnel: [w365] -> w158 mode=indexing
    tunnel: [w353] -> w155 mode=indexing
    tunnel: [w329] -> w100
    w350 = FALSE ("Left")
    n91 = property class="Ctl"(reference=w363, error in=w366) -> (error out=w347:errorcluster, "Label.Text"=w364:string)  [unwired: 1 out]
    n92 = case shown="\"Stage Origin\", Default" w364 {
      tunnel: w347 -> [w369 w377 w389 w394]
      tunnel: [w375 w378 w390 w391] -> w346
      frame "Cam calib" {
        n93 = control-ref of="Spotlights"() -> (w372:refnum<vi>)
        n94 = control-ref of="Coaxial light"() -> (w373:refnum<vi>)
        n95 = call "CheckLightingConditions.vi"("Change Lights? (Change; Coax; Spotlight)"=bool[] [TRUE, TRUE, FALSE], "error in (no error)"=w369, "Spotlights Refnum"=w372, "Coaxial Lights Refnum"=w373) -> ("error out"=w371:errorcluster, "Assigned Camera Gain"=w370:dbl)  [unwired: 4 in, 2 out]
        n96 = property on="Camera gain" class="DigNum (strict)"(error in=w371, "Value"=w370) -> (error out=w376:errorcluster)  [unwired: 1 in, 1 out]
        n97 = call <vilib>:"Simple Error Handler.vi"("error in (no error)"=w376) -> ("error out"=w375:errorcluster)  [unwired: 4 in, 4 out]
      }
      frame "Autofocus" {
        n98 = control-ref of="Spotlights"() -> (w381:refnum<vi>)
        n99 = control-ref of="Coaxial light"() -> (w382:refnum<vi>)
        n100 = call "CheckLightingConditions.vi"("Change Lights? (Change; Coax; Spotlight)"=bool[] [TRUE, TRUE, TRUE], "error in (no error)"=w377, "Spotlights Refnum"=w381, "Coaxial Lights Refnum"=w382) -> ("error out"=w380:errorcluster, "Assigned Camera Gain"=w379:dbl)  [unwired: 4 in, 2 out]
        n101 = property on="Camera gain" class="DigNum (strict)"(error in=w380, "Value"=w379) -> (error out=w378:errorcluster)  [unwired: 1 in, 1 out]
      }
      frame "Bus Tape Circle" {
        n102 = control-ref of="Spotlights"() -> (w384:refnum<vi>)
        n103 = control-ref of="Coaxial light"() -> (w385:refnum<vi>)
        n104 = call "CheckLightingConditions.vi"("Change Lights? (Change; Coax; Spotlight)"=bool[] [TRUE, TRUE, TRUE], "error in (no error)"=w389, "Spotlights Refnum"=w384, "Coaxial Lights Refnum"=w385) -> ("error out"=w388:errorcluster, "Assigned Camera Gain"=w387:dbl)  [unwired: 4 in, 2 out]
        n105 = property on="Camera gain" class="DigNum (strict)"(error in=w388, "Value"=w387) -> (error out=w390:errorcluster)  [unwired: 1 in, 1 out]
      }
      frame "Stage Origin", Default {
        n106 = control-ref of="Spotlights"() -> (w395:refnum<vi>)
        n107 = control-ref of="Coaxial light"() -> (w396:refnum<vi>)
        n108 = call "CheckLightingConditions.vi"("Change Lights? (Change; Coax; Spotlight)"=bool[] [TRUE, TRUE, TRUE], "error in (no error)"=w394, "Spotlights Refnum"=w395, "Coaxial Lights Refnum"=w396) -> ("error out"=w392:errorcluster, "Assigned Camera Gain"=w393:dbl)  [unwired: 4 in, 2 out]
        n109 = property on="Camera gain" class="DigNum (strict)"(error in=w392, "Value"=w393) -> (error out=w391:errorcluster)  [unwired: 1 in, 1 out]
      }
    }
    n110 = Concatenate Strings("Position adjustments queue: " ("name (unnamed)"), w364) -> (w360:string)
    n111 = Concatenate Strings("Checking initial coordinates: " ("Current Build Phase"), w364, "..." ("string")) -> (w345:string)
    n112 = property on="Current Build Phase" class="Str"(error in=w346, "Value"=w345) -> (error out=w341:errorcluster)  [unwired: 1 in, 1 out]
    n113 = property on="Axis Speeds [mm/s]" class="Clust (strict)"(error in=w341) -> (error out=w340:errorcluster, "Value"=w339:cluster{"X":dbl, "Y":dbl, "Z":dbl})  [unwired: 1 in, 1 out]
    n114 = call "Go2XYZ (SubVI).vi"(".NET Refnum in"=w368, "Go to Coordinates"=w367, "Axis Speeds"=w339, "error in (no error)"=w340) -> (".NET Refnum out"=w354:refnum<k24>, "Final Position"=w342:T36, "error out"=w343:errorcluster)  [unwired: 7 in, 2 out]
    "Reset coordinates" <- w342
    n115 = property on="Current stage position [mm]" class="Clust (strict)"(error in=w343, "Value"=w342) -> (error out=w344:errorcluster)  [unwired: 1 in, 1 out]
    n116 = call "AcceptLocationDialogue (SubVI).vi"("error in (no error)"=w344, "Step name"=w364) -> ("error out"=w351:errorcluster, "Accept or Reposition"=w355:bool)  [unwired: 8 in]
    n117 = case shown="True" w355 {
      tunnel: w355 -> [_ w403]
      tunnel: [T27."Enabled" ("Disabled") T27."Disabled and Grayed Out" ("Disabled")] -> w352
      tunnel: w351 -> [w398 w401]
      tunnel: [w398 w400] -> w338
      frame False {
      }
      frame True {
        n118 = property on="Confirm position" class="Bool (strict)"(error in=w401, "Val(Sgnl)"=w403) -> (error out=w400:errorcluster)  [unwired: 1 in, 1 out]
      }
    }
    n119 = property on="Jog step size" class="Clust (strict)"(error in=w338, "DisabledEnum"=w352) -> (error out=w337:errorcluster)  [unwired: 1 in, 1 out]
    n120 = property on="Reset position" class="Bool (strict)"(error in=w338, "DisabledEnum"=w352, "Value"=w350) -> (error out=w332:errorcluster)  [unwired: 1 in, 1 out]
    n121 = property on="Confirm position" class="Bool (strict)"(error in=w338, "DisabledEnum"=w352, "Value"=w350) -> (error out=w331:errorcluster)  [unwired: 1 in, 1 out]
    n122 = property on="Left" class="Bool (strict)"(error in=w338, "DisabledEnum"=w352, "Value"=w350) -> (error out=w336:errorcluster)  [unwired: 1 in, 1 out]
    n123 = property on="Right" class="Bool (strict)"(error in=w338, "DisabledEnum"=w352, "Value"=w350) -> (error out=w335:errorcluster)  [unwired: 1 in, 1 out]
    n124 = property on="Backward" class="Bool (strict)"(error in=w338, "DisabledEnum"=w352, "Value"=w350) -> (error out=w334:errorcluster)  [unwired: 1 in, 1 out]
    n125 = property on="Forward" class="Bool (strict)"(error in=w338, "DisabledEnum"=w352, "Value"=w350) -> (error out=w333:errorcluster)  [unwired: 1 in, 1 out]
    n126 = Merge Errors(w337, w336, w335, w334, w333, w332, w331) -> (w330:errorcluster)
    n127 = Obtain Queue(name (unnamed)=w360, element data type="", error in (no error)=w330) -> (queue out=w359:refnum<queue>, error out=w356:errorcluster)  [unwired: 2 in, 1 out]
    n128 = while "Consumer Loop: Interpret and execute jog instructions" {
      shift-right: [w435] -> _
      shift-left: w359 -> [w436]
      shift-right: [w426] -> _
      shift-left: w356 -> [w434]
      tunnel: w354 -> [w430]
      tunnel: [w418] -> w329
      stop <- w412 stop-if-true
      n129 = Dequeue Element(queue=w436, error in (no error)=w434) -> (queue out=w435:refnum<queue>, element=w428:string, error out=w412:errorcluster)  [unwired: 1 in, 1 out]
      n130 = property on="Axis Speeds [mm/s]" class="Clust (strict)"(error in=w412) -> (error out=w414:errorcluster, "Value"=w422:cluster{"X":dbl, "Y":dbl, "Z":dbl})  [unwired: 1 in, 1 out]
      n131 = property on="Jog step size" class="Clust (strict)"(error in=w412) -> (error out=w415:errorcluster, "Value"=w417:T16)  [unwired: 1 in, 1 out]
      n132 = local read "Reset coordinates"() -> (w433:cluster{"X":dbl, "Y":dbl, "Z":dbl})
      n133 = Merge Errors(w414, w415) -> (w413:errorcluster)
      n134 = call "JogStepInterpeter (SubVI).vi"("Jog step size ENUM"=w417) -> ("Jog step size"=w416:T37)
      n135 = call "XYZToggleJog (SubVI).vi"("Aerotech in"=w430, "Motion direction"=w428, "Start location"=w433, "Jog step size"=w416, "Axis Speeds"=w422, "error in (no error)"=w413) -> ("Aerotech out"=w418:refnum<k24>, "Current stage position [mm]"=w423:cluster{"X":dbl, "Y":dbl, "Z":dbl}, "completed"=w429:bool, "error out"=w425:errorcluster)  [unwired: 5 in, 1 out]
      n136 = property on="Current stage position [mm]" class="Clust (strict)"(error in=w425, "Value"=w423) -> (error out=w424:errorcluster)  [unwired: 1 in, 1 out]
      n137 = Not(x=w429) -> (.not. x?=w427:bool)
      n138 = case shown="\"-X\"" w428 {
        tunnel: w427 -> [w437 w440 w445 w447 w450 w453 _]
        tunnel: w424 -> [w438 w441 w444 w448 w451 w454 w455]
        tunnel: [w439 w442 w443 w446 w449 w452 w455] -> w409
        frame "-X" {
          n139 = property on="Left" class="Bool (strict)"(error in=w438, "Value"=w437) -> (error out=w439:errorcluster)  [unwired: 1 in, 1 out]
        }
        frame "X" {
          n140 = property on="Right" class="Bool (strict)"(error in=w441, "Value"=w440) -> (error out=w442:errorcluster)  [unwired: 1 in, 1 out]
        }
        frame "-Y" {
          n141 = property on="Forward" class="Bool (strict)"(error in=w444, "Value"=w445) -> (error out=w443:errorcluster)  [unwired: 1 in, 1 out]
        }
        frame "Y" {
          n142 = property on="Backward" class="Bool (strict)"(error in=w448, "Value"=w447) -> (error out=w446:errorcluster)  [unwired: 1 in, 1 out]
        }
        frame "ALL" {
          n143 = property on="Reset position" class="Bool (strict)"(error in=w451, "Value"=w450) -> (error out=w449:errorcluster)  [unwired: 1 in, 1 out]
        }
        frame "DONE" {
          n144 = property on="Confirm position" class="Bool (strict)"(error in=w454, "Value"=w453) -> (error out=w452:errorcluster)  [unwired: 1 in, 1 out]
        }
        frame "NULL", Default {
        }
      }
      n145 = property on="Current stage position [mm]" class="Clust (strict)"(error in=w409) -> (error out=w410:errorcluster, "Value"=w421:cluster{"X":dbl, "Y":dbl, "Z":dbl})  [unwired: 1 in, 1 out]
      n146 = property on="Jog step size" class="Clust (strict)"(error in=w409) -> (error out=w408:errorcluster, "Value"=w420:T16)  [unwired: 1 in, 1 out]
      n147 = control-ref of="Left"() -> (w432:refnum<vi>)
      n148 = control-ref of="Forward"() -> (w405:refnum<vi>)
      n149 = control-ref of="Up"() -> (w407:refnum<vi>)
      n150 = control-ref of="Right"() -> (w431:refnum<vi>)
      n151 = control-ref of="Backward"() -> (w404:refnum<vi>)
      n152 = control-ref of="Down"() -> (w406:refnum<vi>)
      n153 = Merge Errors(w410, w408) -> (w411:errorcluster)
      n154 = call "JogStepInterpeter (SubVI).vi"("Jog step size ENUM"=w420) -> ("Jog step size"=w419:T37)
      n155 = call "ActivateToggleControls (SubVI).vi"("Left refnum"=w432, "Current stage position [mm]"=w421, "Right refnum"=w431, "Forward refnum"=w405, "Backward refnum"=w404, "error in (no error)"=w411, "Jog step size"=w419, "Up refnum"=w407, "Down refnum"=w406) -> ("error out"=w426:errorcluster)  [unwired: 6 in]
    }
    n156 = while "Producer Loop: Collect jog input instructions" {
      shift-right: [w471] -> w357
      shift-left: w356 -> [w463]
      shift-right: [w470] -> w358
      shift-left: w359 -> [w475]
      tunnel: [w469] -> w365
      stop <- w473 stop-if-true
      # "Up/Down disabled! They are not fully implemented. See Utils/Standalone/ContinuousStageAndCamera\nto see their full implementation"
      n157 = control-ref of="Down"() -> (w458:refnum<vi>)
      n158 = property on="Current stage position [mm]" class="Clust (strict)"(error in=w463) -> (error out=w462:errorcluster, "Value"=w464:cluster{"X":dbl, "Y":dbl, "Z":dbl})  [unwired: 1 in, 1 out]